vi "OFDM_Tx_5.0.vi"() -> ()   [LabVIEW 2015]
uses:
  <vilib>/Analysis/2dsp.llb/Inverse Complex FFT.vi
  <vilib>/addons/Modulation/Digital/General/MT Generate QAM System Parameters(M).vi
  <vilib>/addons/Modulation/Digital/General/MT Map Bits to QAM Symbols.vi
  <vilib>/imath/engines/lvmath2/RunTimeEngine/RangeToken/NIMS_Range.vi
  <instcachedir>/0/NIMS_Range_D919CC09935940E88F755EC1C6F49AC1.lvgen/NIMS_Range_D919CC09935940E88F755EC1C6F49AC1_001.vi
  <vilib>/imath/engines/lvmath2/RunTimeEngine/BuiltInFunctions/sets_diff/NIMS_sets_diff(GV2).vi
  <instcachedir>/0/NIMS_sets_diff(GV2)_CE188B9DAFCC49368CD9C62F83DF72AA.lvgen/NIMS_sets_diff(GV2)_CE188B9DAFCC49368CD9C62F83DF72AA_007.vi
  <vilib>/imathl/engines/lvmath/Functions/Error Handling/Create Error.vi
  <vilib>/imath/engines/lvmath2/RunTimeEngine/BuiltInFunctions/rand/NIMS_rand(1,I32).vi
  <vilib>/imath/engines/lvmath2/RunTimeEngine/ErrorHandling/NIMS_Error From Error Code.vi
  <vilib>/imath/engines/lvmath2/RunTimeEngine/IndexReplace/NIMS V(V)=V.vi
  <instcachedir>/0/NIMS V(V)=V_422D7BAD0B0F4E4DA085EB3347135799.lvgen/NIMS V(V)=V_422D7BAD0B0F4E4DA085EB3347135799_000.vi
  <vilib>/imath/engines/lvmath2/RunTimeEngine/IndexRead/NIMS V(R2).vi
  <instcachedir>/0/NIMS V(R2)_C76619605A0E4E9F8B2FA9389712AC47.lvgen/NIMS V(R2)_C76619605A0E4E9F8B2FA9389712AC47_002.vi
  <instcachedir>/0/NIMS V(R2)_C76619605A0E4E9F8B2FA9389712AC47.lvgen/NIMS V(R2)_C76619605A0E4E9F8B2FA9389712AC47_001.vi
  <instcachedir>/0/NIMS V(V)=V_422D7BAD0B0F4E4DA085EB3347135799.lvgen/NIMS V(V)=V_422D7BAD0B0F4E4DA085EB3347135799_001.vi
  <vilib>/imath/engines/lvmath2/RunTimeEngine/ErrorHandling/NIMS_Create Error From Enums.vi
  <vilib>/imath/engines/lvmath2/RunTimeEngine/NodeEndStatement/NIMS_NodeEndStatement_Output.vi
  <instcachedir>/0/NIMS_NodeEndStatement_Output_53EC0D466D134D7ABD903AC30B43404B.lvgen/NIMS_NodeEndStatement_Output_53EC0D466D134D7ABD903AC30B43404B_010.vi
  <instcachedir>/0/NIMS_NodeEndStatement_Output_53EC0D466D134D7ABD903AC30B43404B.lvgen/NIMS_NodeEndStatement_Output_53EC0D466D134D7ABD903AC30B43404B_000.vi
  <vilib>/imath/engines/lvmath2/RunTimeEngine/ErrorHandling/NIMS_Finalize Error.vi
  <instrlib>/niUSRP/niUSRP Write Tx Data (CDB).vi
  <vilib>/addons/Modulation/niDMT.lvlib
  <vilib>/Analysis/NI_AALPro.lvlib
panel:
  out "TX Output":cdb[](array[numeric])
  out "Bit Stream":i8[](array[numeric])
  out "num_frames":i64=8
  in  "cp_length":i16=28
  in  "frame_length":i64=220
  in  "pilot_offset_time":i16=4
  in  "pilot_offset_freq":i16=12
  in  "pilot_start":i16=2
  in  "SC_pilot":i16=18
  in  "SC_data":i64=180
  in  "SC_total":i16=256
  in  "Symbol Rate (sym/sec)":i16=10000
  out "coerced gain":dbl=3.0 format="%#_6f"
  out "coerced carrier frequency":dbl=2422000000.004802 format="%#_6p"
  out "coerced IQ rate":dbl=7692307.692307692 format="%#_6p"
  in  "?":bool
  out "error out":errorcluster
  in  "IQ rate":dbl=8000000.0 format="%#_6p"
  in  "Gain (dB)":dbl=3.0 format="%#_6f"
  in  "TX Antenna":string="TX1"
  in  "Carrier Frequency (Hz)":dbl=2422000000.0 format="%#_6p"
  in  "TX Device":refnum<k15>="192.168.10.2"
  # "USRP PARAMETERS"
  # "OFDM PARAMETERS"
  # "PILOT DISTRIBUTION PARAMETERS"
  # "INDICATORS"
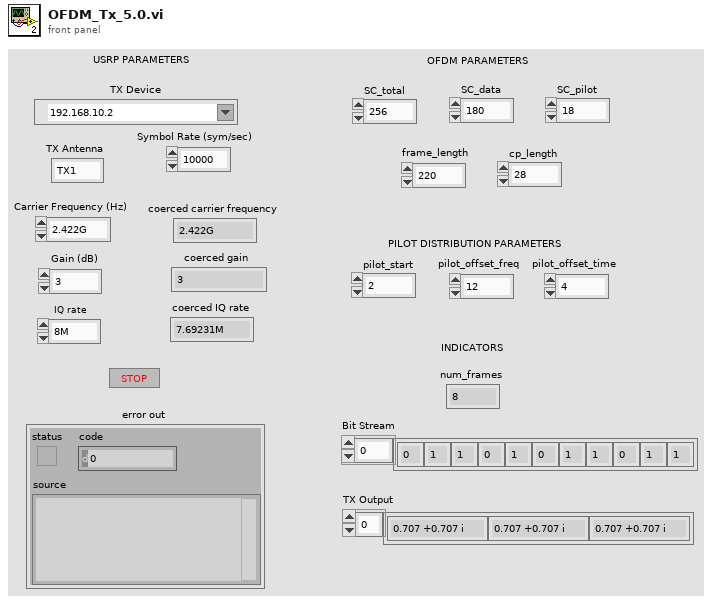
[diagram p1: front panel]
types:
  T1 = cluster{"samples per symbol (16)":i32, "symbol map":cdb[]}
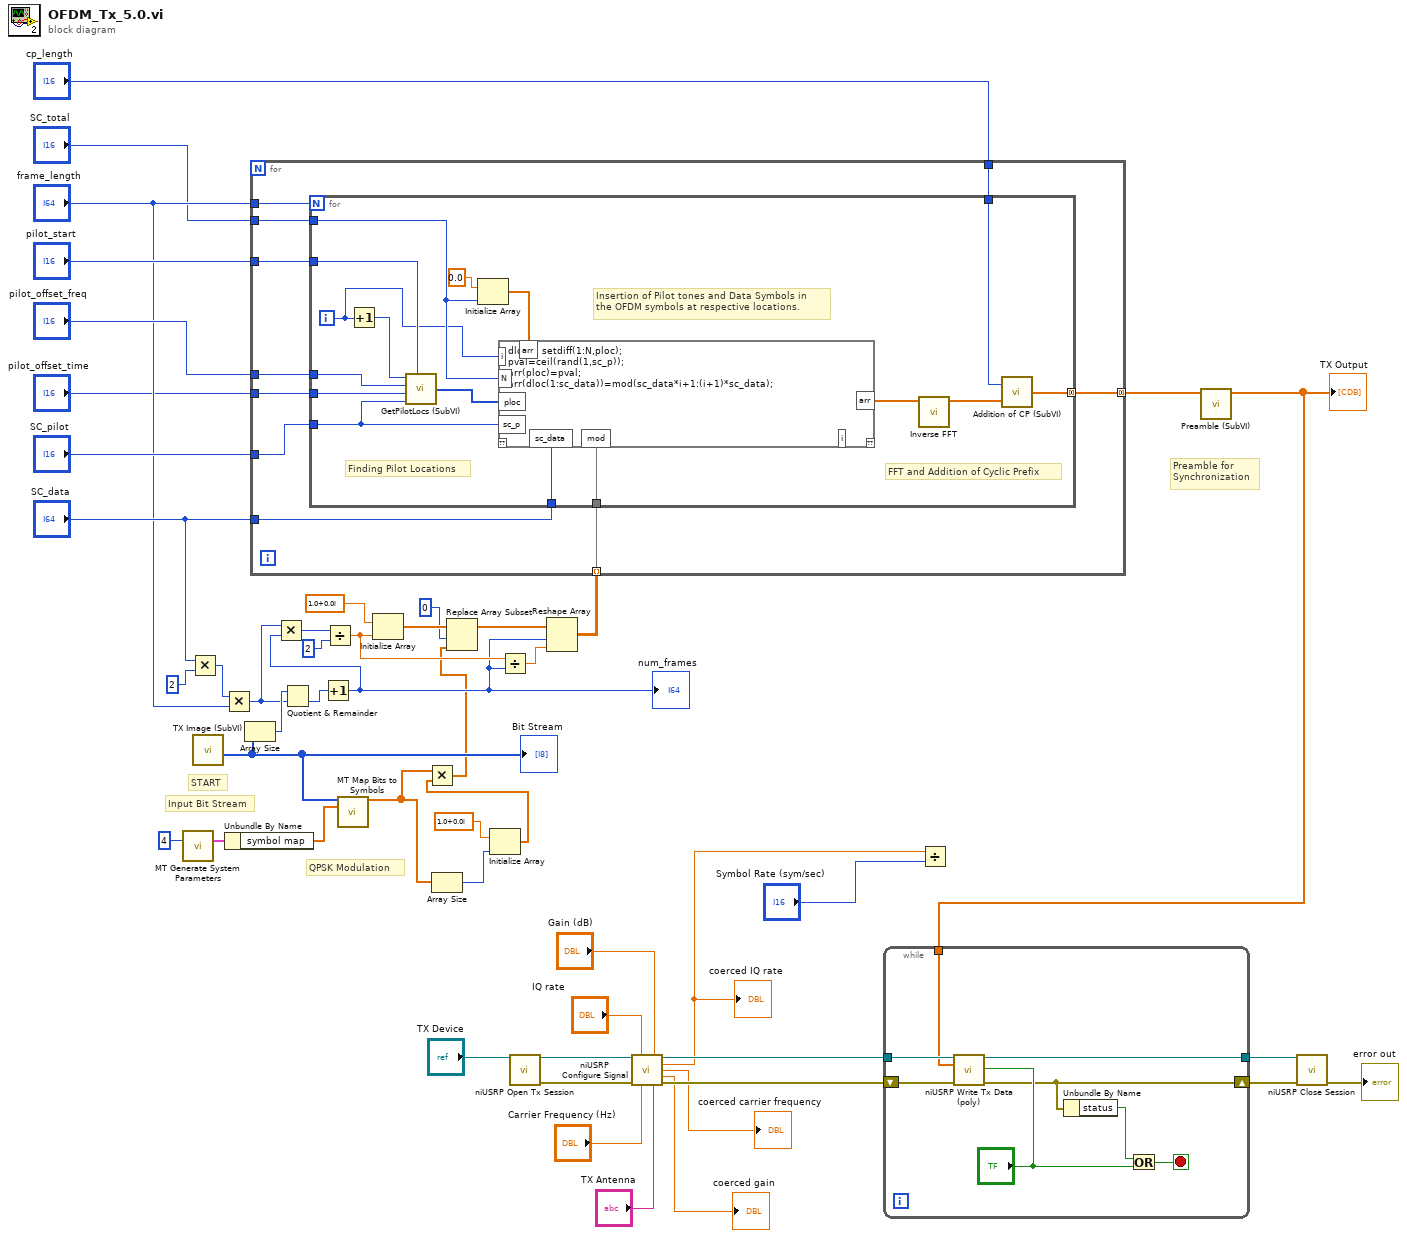
[diagram p0: block diagram]
diagram:
  # "Preamble for\nSynchronization"
  # "START"
  # "Input Bit Stream"
  # "QPSK Modulation"
  n1 = call-poly <vilib>:"MT Generate System Parameters.vi"("M-QAM (16)"=4) -> ("QAM system parameters"=w33:T1)  [unwired: 12 in, 2 out]
  n2 = Multiply(x="SC_data", y=i64 2) -> (x*y=w25:i64)
  n3 = call "TX Image (SubVI).vi"() -> ("image_bits"=w10:i8[])  [unwired: 9 in, 2 out]
  "Bit Stream" <- w10
  n4 = Multiply(x=w25, y="frame_length") -> (x*y=w22:i64)
  n5 = Unbundle By Name(w33) -> ("symbol map"=w32:cdb[])
  n6 = Array Size(array=w10) -> (size(s)=w24:i32)
  n7 = Quotient & Remainder(x=w24, y=w22) -> (floor(x/y)=w23:i64)  [unwired: 1 out]
  n8 = Increment(x=w23) -> (x+1=w12:i64)
  "num_frames" <- w12
  n9 = Multiply(x=w22, y=w12) -> (x*y=w18:i64)
  n10 = Divide(x=w18, y=i64 2 ("x")) -> (x/y=w15:dbl)
  n11 = call-poly <vilib>:"MT Map Bits to Symbols.vi"("input bit stream"=w10, "symbol map"=w32) -> ("symbols"=w4:cdb[])  [unwired: 12 in, 1 out]
  n12 = Initialize Array(cdb 1.0+0.0i ("element"), w15) -> (w21:cdb[])
  n13 = Array Size(array=w4) -> (size(s)=w6:i32)
  n14 = Initialize Array(cdb 1.0+0.0i ("element"), w6) -> (w5:cdb[])
  n15 = Multiply(x=w4, y=w5) -> (x*y=w3:cdb[])
  n16 = Replace Array Subset(array=w21, new element=w3, index=0) -> (w16:cdb[])
  n17 = Divide(x=w15, y=w12) -> (x/y=w14:dbl)
  n18 = call <instrlib>:"niUSRP Open Tx Session.vi"("device names"="TX Device") -> ("session handle out"=w49:refnum<k15>, "error out"=w48:errorcluster)  [unwired: 13 in]
  n19 = Reshape Array(w16, w12, w14) -> (w13:cdb[][])
  n20 = for {
    tunnel: "cp_length" -> [w60]
    tunnel: "SC_total" -> [w59]
    tunnel: "pilot_start" -> [w58]
    tunnel: "pilot_offset_freq" -> [w57]
    tunnel: "pilot_offset_time" -> [w56]
    tunnel: [w55] -> w1 mode=concatenating
    tunnel: "SC_pilot" -> [w51]
    tunnel: "SC_data" -> [w54]
    tunnel: "frame_length" -> [w53]
    tunnel: w13 -> [w52] mode=indexing
    n21 = for {
      N: w53 -> [_]
      tunnel: w56 -> [w76]
      tunnel: w57 -> [w75]
      tunnel: w58 -> [w74]
      tunnel: w51 -> [w61]
      tunnel: w59 -> [w67]
      tunnel: w54 -> [w65]
      tunnel: w52 -> [w64]
      tunnel: w60 -> [w63]
      tunnel: [w62] -> w55 mode=concatenating
      i -> [w66]
      # "FFT and Addition of Cyclic Prefix"
      # "Insertion of Pilot tones and Data Symbols in \nthe OFDM symbols at respective locations."
      # "Finding Pilot Locations"
      n22 = Increment(x=w66) -> (x+1=w68:i32)
      n23 = call "GetPilotLocs (SubVI).vi"("sym #"=w68, "pilot_offset_freq"=w75, "pilot_offset_time"=w76, "sc_pilot"=w61, "pilot_start"=w74) -> ("Array"=w73:i32[])
      n24 = Initialize Array(0.0 ("element"), w67) -> (w71:dbl[])
      n25 = mathscript code="dloc = setdiff(1:N,ploc);\npval=ceil(rand(1,sc_p));\narr(ploc)=pval;\narr(dloc(1:sc_data))=mod(sc_data*i+1:(i+1)*sc_data);"("ploc"=w73, "N"=w67, "arr"=w71, "sc_p"=w61, "mod"=w64, "sc_data"=w65, "i"=w66) -> ("arr"=w70:cdb[])  [unwired: 1 in, 2 out]
      n26 = call-poly <vilib>:"Inverse FFT.vi"("FFT {X}"=w70) -> ("X"=w69:cdb[])  [unwired: 9 in, 1 out]
      n27 = call "Addition of CP (SubVI).vi"("ifft_output"=w69, "cp_length"=w63) -> ("ifft_output with CP"=w62:cdb[])
    }
  }
  n28 = call <instrlib>:"niUSRP Configure Signal.vi"("session handle"=w49, "IQ rate"="IQ rate", "carrier frequency"="Carrier Frequency (Hz)", "gain"="Gain (dB)", "error in (no error)"=w48, "active antenna"="TX Antenna") -> ("session handle out"=w39:refnum<k15>, "coerced IQ rate"=w35:dbl, "coerced carrier frequency"=→"coerced carrier frequency":dbl, "coerced gain"=→"coerced gain":dbl, "error out"=w43:errorcluster)  [unwired: 5 in]
  "coerced IQ rate" <- w35
  n29 = Divide(x=w35, y="Symbol Rate (sym/sec)") -> ()  [unwired: 1 out]
  n30 = call "Preamble (SubVI).vi"("array in"=w1) -> ("array out"=w2:cdb[])  [unwired: 10 in]
  "TX Output" <- w2
  n31 = while {
    shift-right: [w215] -> w41
    shift-left: w43 -> [w220]
    tunnel: w39 -> [w218]
    tunnel: [w219] -> w42
    tunnel: w2 -> [w213]
    stop <- w217 stop-if-true
    n32 = call-poly <instrlib>:"niUSRP Write Tx Data (poly).vi"("session handle"=w218, "data"=w213, "end of data?"="?", "error in (no error)"=w220) -> ("session handle out"=w219:refnum<k15>, "error out"=w215:errorcluster)  [unwired: 10 in]
    n33 = Unbundle By Name(w215) -> ("status"=w214:bool)
    n34 = Or(x=w214, y="?") -> (x .or. y?=w217:bool)
  }
  n35 = call <instrlib>:"niUSRP Close Session.vi"("session handle"=w42, "error in (no error)"=w41) -> ("error out"=→"error out":errorcluster)  [unwired: 13 in]
